vi "HFRR ADV v040.vi"() -> ()   [LabVIEW 2025] (continued)
        n290 = Format Into String(format string="%<%I:%M:%S:%p %d:%B:%Y>T", w374) -> (resulting string=→"Time Stamp":string)  [unwired: 2 in, 1 out]
        n291 = local read "Service Password enable"() -> (w366:bool)
        n292 = local read "FILE"() -> (w371:string)
        n293 = call <vilib>:"Trim Whitespace.vi"("string"=w371) -> ("trimmed string"=w370:string)  [unwired: 1 in]
        n294 = String Length(string=w370) -> (length=w369:i32)
        n295 = Greater?(x=w369, y=1) -> (0:w367:bool)
        n296 = case shown="False" w367 {
          tunnel: w366 -> [w395 _]
          frame False {
            n297 = case shown="False" w395 {
              frame True {
                w396 = "Test Start In Service Mode" ("Tip Strip")
                w397 = T19."Enabled" ("Disabled")
                n298 = property on="Auto Start Test" class="Bool (strict)"("DisabledEnum"=w397, "TipStrip"=w396) -> ()  [unwired: 2 in, 2 out]
                n299 = property on="RUN" class="Bool (strict)"("DisabledEnum"=w397, "TipStrip"=w396) -> ()  [unwired: 2 in, 2 out]
              }
              frame False {
                w398 = "Enter File Name to Start Test" ("Tip Strip")
                w399 = T19."Disabled and Grayed Out" ("Disabled")
                n300 = property on="Auto Start Test" class="Bool (strict)"("DisabledEnum"=w399, "TipStrip"=w398) -> ()  [unwired: 2 in, 2 out]
                n301 = property on="RUN" class="Bool (strict)"("DisabledEnum"=w399, "TipStrip"=w398) -> ()  [unwired: 2 in, 2 out]
              }
            }
          }
          frame True {
            w400 = "" ("Tip Strip")
            w401 = T19."Enabled" ("Disabled")
            n302 = property on="Auto Start Test" class="Bool (strict)"("DisabledEnum"=w401, "TipStrip"=w400) -> ()  [unwired: 2 in, 2 out]
            n303 = property on="RUN" class="Bool (strict)"("DisabledEnum"=w401, "TipStrip"=w400) -> ()  [unwired: 2 in, 2 out]
          }
        }
      }
      event "RUN": Value Change {
        n304 = event-data() -> ()  [unwired: 1 in, 6 out]
        n305 = local read "RUN"() -> (w403:bool)
        n306 = case shown="False" w403 {
          frame False {
            n307 = flat-sequence {
              frame #0 {
                n308 = local write "START TEMP"(FALSE ("START TEMP")) -> ()
              }
              frame #1 {
                n309 = Wait (ms)(milliseconds to wait=u32 1500) -> ()  [unwired: 1 out]
              }
              frame #2 {
                n310 = local write "Humidity 2"(TRUE ("Humidity")) -> ()
              }
              frame #3 {
                n311 = local write "Due Write"("VC;0") -> ()
              }
              frame #4 {
                n312 = Wait (ms)(milliseconds to wait=u32 1500) -> ()  [unwired: 1 out]
              }
              frame #5 {
                w413 = T19."Enabled" ("Disabled")
                (unwired) T26."Imaging" ("Main Dashboard Buttons")
                (unwired) T21."Adv Scar" ("Main Tab")
                w415 = "" ("FILE")
                n313 = local write "measured_stroke"(0.0 ("measured_stroke")) -> ()
                n314 = local write "Due Write"("VC;0") -> ()
                n315 = local write "FILE"(w415) -> ()
                n316 = local write "Batch Ref Num :"(w415) -> ()
                n317 = local write "Fuel Discription :"(w415) -> ()
                n318 = local write "Main Tab"(T2."Adv Scar" ("Main Tab")) -> ()
                n319 = local write "Remarks :"(w415) -> ()
                n320 = local write "Main Dashboard Buttons"(T1."Imaging" ("Main Dashboard Buttons")) -> ()
                n321 = local write "TEST FILE NAM,E SAVED"(FALSE ("TEST FILE NAM,E SAVED")) -> ()
                n322 = property on="Stroke ( mm )" class="WFChart (strict)"("History Data"=cluster{"y":dbl, dbl, "y":dbl}[] []) -> ()  [unwired: 2 in, 2 out]
                n323 = property on="Auto Start Test" class="Bool (strict)"("Visible"=TRUE) -> ()  [unwired: 2 in, 2 out]
                n324 = property on="FRICVALZ 2" class="Bool (strict)"("DisabledEnum"=w413) -> ()  [unwired: 2 in, 2 out]
                n325 = property on="FRICVALZ 4" class="Bool (strict)"("DisabledEnum"=w413) -> ()  [unwired: 2 in, 2 out]
                n326 = property on="FRICVALZ 3" class="Bool (strict)"("DisabledEnum"=w413) -> ()  [unwired: 2 in, 2 out]
              }
            }
          }
          frame True {
            n327 = stacked-sequence {
              frame #0 {
                n328 = local write "Due Write"("DAC;200") -> ()
              }
              frame #1 {
                n329 = Wait (ms)(milliseconds to wait=u32 1500) -> ()  [unwired: 1 out]
              }
              frame #2 {
                n330 = local write "Due Write"("DAC;200") -> ()
              }
              frame #3 {
                n331 = Wait (ms)(milliseconds to wait=u32 1500) -> ()  [unwired: 1 out]
              }
              frame #4 {
                n332 = local write "Due Write"("VC;1") -> ()
              }
              frame #5 {
                n333 = Wait (ms)(milliseconds to wait=u32 2000) -> ()  [unwired: 1 out]
              }
              frame #6 {
                n334 = local write "Due Write"("VC;1") -> ()
              }
              frame #7 {
                n335 = Wait (ms)(milliseconds to wait=u32 2000) -> ()  [unwired: 1 out]
              }
              frame #8 {
                w427 = T19."Disabled" ("Disabled")
                n336 = property on="Auto Start Test" class="Bool (strict)"("Visible"=FALSE) -> ()  [unwired: 2 in, 2 out]
                n337 = local write "START TEMP"(TRUE ("START TEMP")) -> ()
                n338 = property on="FRICVALZ 2" class="Bool (strict)"("DisabledEnum"=w427) -> ()  [unwired: 2 in, 2 out]
                n339 = property on="FRICVALZ 4" class="Bool (strict)"("DisabledEnum"=w427) -> ()  [unwired: 2 in, 2 out]
                n340 = property on="FRICVALZ 3" class="Bool (strict)"("DisabledEnum"=w427) -> ()  [unwired: 2 in, 2 out]
              }
            }
          }
        }
      }
      event "run test Calibration": Value Change {
        n341 = event-data() -> ()  [unwired: 1 in, 6 out]
        n342 = local read "run test Calibration"() -> (w429:bool)
        n343 = case shown="True" w429 {
          frame False {
            n344 = flat-sequence {
              frame #0 {
                n345 = local write "START TEMP"(FALSE ("START TEMP")) -> ()
              }
              frame #1 {
                n346 = Wait (ms)(milliseconds to wait=u32 1500) -> ()  [unwired: 1 out]
              }
              frame #2 {
              }
              frame #3 {
                n347 = local write "Due Write"("VC;0") -> ()
              }
              frame #4 {
                n348 = Wait (ms)(milliseconds to wait=u32 1500) -> ()  [unwired: 1 out]
              }
              frame #5 {
                n349 = local write "Due Write"("VC;0") -> ()
              }
            }
          }
          frame True {
            n350 = flat-sequence {
              frame #0 {
                n351 = local write "Due Write"("VC;1") -> ()
              }
              frame #1 {
                n352 = Wait (ms)(milliseconds to wait=u32 2000) -> ()  [unwired: 1 out]
              }
              frame #2 {
                n353 = local write "Due Write"("VC;1") -> ()
              }
              frame #3 {
                n354 = Wait (ms)(milliseconds to wait=u32 2000) -> ()  [unwired: 1 out]
              }
              frame #4 {
                n355 = local write "START TEMP"(TRUE ("START TEMP")) -> ()
              }
            }
          }
        }
      }
      event "Auto": Value Change {
        n356 = event-data() -> ()  [unwired: 1 in, 6 out]
        n357 = stacked-sequence {
          frame #0 {
            n358 = local write "FILE"("") -> ()
          }
          frame #1 {
            n359 = Get Date/Time In Seconds() -> (seconds since 1Jan1904=w445:timestamp)
            n360 = Format Into String(format string="%<%I_%M_%S_%p_%d_%B_%Y>T", w445) -> (resulting string=w444:string)  [unwired: 2 in, 1 out]
            n361 = local write "FILE"(w444) -> ()
          }
        }
        n362 = local read "Auto"() -> (w442:bool)
        n363 = Not(x=w442) -> (.not. x?=w441:bool)
        n364 = local write "Auto"(w441) -> ()
      }
      event "Auto Start Temp": Value Change {
        n365 = event-data() -> ()  [unwired: 1 in, 6 out]
        n366 = local read "Auto Start Test"() -> (w448:bool)
        n367 = case shown="False" w448 {
          frame False {
            n368 = stacked-sequence {
              frame #0 {
                n369 = local write "START TEMP"(FALSE ("START TEMP")) -> ()
              }
              frame #1 {
                n370 = Wait (ms)(milliseconds to wait=u32 2000) -> ()  [unwired: 1 out]
              }
              frame #2 {
                n371 = local write "Due Write"("VC;0") -> ()
              }
              frame #3 {
                n372 = Wait (ms)(milliseconds to wait=u32 2000) -> ()  [unwired: 1 out]
              }
              frame #4 {
                w459 = T19."Enabled" ("Disabled")
                (unwired) T26."Imaging" ("Main Dashboard Buttons")
                w460 = "" ("FILE")
                n373 = local write "Main Tab"(T2."Adv Scar" ("Main Tab")) -> ()
                n374 = local write "measured_stroke"(0.0 ("measured_stroke")) -> ()
                n375 = local write "Main Dashboard Buttons"(T1."Imaging" ("Main Dashboard Buttons")) -> ()
                n376 = property on="RUN" class="Bool (strict)"("Visible"=TRUE) -> ()  [unwired: 2 in, 2 out]
                n377 = local write "Due Write"("VC;0") -> ()
                n378 = local write "Humidity 2"(TRUE ("Humidity")) -> ()
                n379 = local write "TEST FILE NAM,E SAVED"(FALSE ("TEST FILE NAM,E SAVED")) -> ()
                n380 = local write "Fuel Discription :"(w460) -> ()
                n381 = local write "Batch Ref Num :"(w460) -> ()
                n382 = local write "Remarks :"(w460) -> ()
                n383 = local write "FILE"(w460) -> ()
                n384 = property on="FRICVALZ 2" class="Bool (strict)"("DisabledEnum"=w459) -> ()  [unwired: 2 in, 2 out]
                n385 = property on="FRICVALZ 4" class="Bool (strict)"("DisabledEnum"=w459) -> ()  [unwired: 2 in, 2 out]
                n386 = property on="FRICVALZ 3" class="Bool (strict)"("DisabledEnum"=w459) -> ()  [unwired: 2 in, 2 out]
              }
            }
          }
          frame True {
            n387 = stacked-sequence {
              frame #0 {
                n388 = local write "Due Write"("DAC;200") -> ()
              }
              frame #1 {
                n389 = Wait (ms)(milliseconds to wait=u32 1500) -> ()  [unwired: 1 out]
              }
              frame #2 {
                n390 = local write "Due Write"("DAC;200") -> ()
              }
              frame #3 {
                n391 = Wait (ms)(milliseconds to wait=u32 1000) -> ()  [unwired: 1 out]
              }
              frame #4 {
                n392 = local write "Due Write"("VC;1") -> ()
              }
              frame #5 {
                n393 = Wait (ms)(milliseconds to wait=u32 2000) -> ()  [unwired: 1 out]
              }
              frame #6 {
                n394 = local write "Due Write"("VC;1") -> ()
              }
              frame #7 {
                n395 = Wait (ms)(milliseconds to wait=u32 2000) -> ()  [unwired: 1 out]
              }
              frame #8 {
                w471 = T19."Disabled" ("Disabled")
                n396 = property on="RUN" class="Bool (strict)"("Visible"=FALSE) -> ()  [unwired: 2 in, 2 out]
                n397 = property on="FRICVALZ 2" class="Bool (strict)"("DisabledEnum"=w471) -> ()  [unwired: 2 in, 2 out]
                n398 = property on="FRICVALZ 4" class="Bool (strict)"("DisabledEnum"=w471) -> ()  [unwired: 2 in, 2 out]
                n399 = property on="FRICVALZ 3" class="Bool (strict)"("DisabledEnum"=w471) -> ()  [unwired: 2 in, 2 out]
                "START TEMP" <- TRUE
              }
            }
          }
        }
      }
      event "FILE", "USERNAME", "USER ID": Mouse Enter {
        n400 = event-data() -> ()  [unwired: 1 in, 4 out]
        n401 = dll-call lib="kernel32.dll" fn="Wow64DisableWow64FsRedirection"("OldValue"=0) -> (error out=w478:errorcluster, "OldValue"=w476:i32)  [unwired: 4 in, 1 out]
        n402 = call <vilib>:"System Exec.vi"("run minimized? (F)"=TRUE, "error in (no error)"=w478, "command line"="C:\\Program Files\\Common Files\\Microsoft Shared\\Ink\\TabTip.exe") -> ("error out"=w477:errorcluster)  [unwired: 5 in, 3 out]
        n403 = dll-call lib="kernel32.dll" fn="Wow64EnableWow64FsRedirection"(error in=w477, "OldValue"=w476) -> ()  [unwired: 4 in, 2 out]
      }
      event "EDIT": Value Change {
        n404 = event-data() -> ()  [unwired: 1 in, 6 out]
        n405 = local read "EDIT"() -> (w479:bool)
        n406 = case shown="False" w479 {
          frame False {
            n407 = control-ref of="This VI"() -> (w496:refnum<vi>)
            n408 = property class="VI"(reference=w496) -> (reference out=w487:refnum<vi>, error out=w491:errorcluster, "Panel"=w495:refnum<vi>)  [unwired: 1 in]
            n409 = property class="Pnl"(reference=w495, error in=w491) -> (reference out=w489:refnum<vi>, error out=w492:errorcluster, "Panes[]"=w494:refnum<vi>[])
            n410 = for {
              tunnel: w494 -> [w502] mode=indexing
              tunnel: T24."Always Off" ("Horizontal Scrollbar Visibility") -> [w501]
              tunnel: w492 -> [w498]
              tunnel: [w497] -> w490
              n411 = property class="Pane"(reference=w502, error in=w498, "HorizScrollbarVisibility"=w501) -> (reference out=w499:refnum<vi>, error out=w500:errorcluster)
              n412 = Close Reference(reference=w499, error in (no error)=w500) -> (error out=w497:errorcluster)
            }
            n413 = Close Reference(reference=w489, error in (no error)=w490) -> (error out=w488:errorcluster)
            n414 = Close Reference(reference=w487, error in (no error)=w488) -> (error out=w482:errorcluster)
            "error out 7" <- w482
            n415 = call <vilib>:"Clear Errors.vi"("error in (no error)"=w482) -> ("error out"=w481:errorcluster)  [unwired: 5 in, 1 out]
            n416 = local write "Service Password enable"(FALSE ("Service Password enable")) -> ()
            n417 = call <userlib>:"Fit VI window to Largest Dec.vi"("error in (no error)"=w481, "border spacing (2 px)"=1) -> ("error out"=w486:errorcluster, "dup VI Ref"=w484:refnum<vi>)  [unwired: 4 in]
            n418 = invoke on="Invoke Node" class="VI" method="FP.Run-Time Position.Maximized"(reference=w484, error in=w486) -> (error out=w485:errorcluster)  [unwired: 2 in, 3 out]
            n419 = call <vilib>:"Clear Errors.vi"("error in (no error)"=w485) -> ()  [unwired: 5 in, 2 out]
          }
          frame True {
          }
        }
      }
      event "Heater Button": Value Change {
        n420 = event-data() -> ()  [unwired: 1 in, 6 out]
        n421 = local read "Heater Button"() -> (w503:bool)
        n422 = case shown="True" w503 {
          frame True {
            n423 = stacked-sequence {
              frame #0 {
                n424 = Wait (ms)(milliseconds to wait=u32 1500) -> ()  [unwired: 1 out]
              }
              frame #1 {
                n425 = local read "Set Temp"() -> (w505:dbl)
                n426 = Number To Fractional String(number=w505, precision (6)=i16 2) -> (F-format string=w508:string)  [unwired: 2 in]
                n427 = Concatenate Strings("ST;" ("Command"), w508) -> (w507:string)
                n428 = local write "Due Write"(w507) -> ()
              }
              frame #2 {
                n429 = Wait (ms)(milliseconds to wait=u32 1500) -> ()  [unwired: 1 out]
              }
              frame #3 {
                n430 = local write "Due Write"("HE;1" ("Command")) -> ()
              }
              frame #4 {
                n431 = Wait (ms)(milliseconds to wait=u32 1500) -> ()  [unwired: 1 out]
              }
              frame #5 {
                n432 = stacked-sequence {
                  frame #0 {
                    n433 = Wait (ms)(milliseconds to wait=u32 1500) -> ()  [unwired: 1 out]
                  }
                  frame #1 {
                    n434 = local read "Set Temp"() -> (w514:dbl)
                    n435 = Number To Fractional String(number=w514, precision (6)=i16 2) -> (F-format string=w517:string)  [unwired: 2 in]
                    n436 = Concatenate Strings("ST;" ("Command"), w517) -> (w516:string)
                    n437 = local write "Due Write"(w516) -> ()
                  }
                  frame #2 {
                    n438 = Wait (ms)(milliseconds to wait=u32 1500) -> ()  [unwired: 1 out]
                  }
                  frame #3 {
                    n439 = local write "Due Write"("HE;1" ("Command")) -> ()
                  }
                  frame #4 {
                    n440 = Wait (ms)(milliseconds to wait=u32 1500) -> ()  [unwired: 1 out]
                  }
                }
              }
            }
          }
          frame False {
            n441 = stacked-sequence {
              frame #0 {
                n442 = Wait (ms)(milliseconds to wait=u32 1500) -> ()  [unwired: 1 out]
              }
              frame #1 {
                n443 = Concatenate Strings("ST;" ("Command"), "0" ("string")) -> (w524:string)
                n444 = local write "Due Write"(w524) -> ()
              }
              frame #2 {
                n445 = Wait (ms)(milliseconds to wait=u32 1500) -> ()  [unwired: 1 out]
              }
              frame #3 {
                n446 = local write "Due Write"("HE;0" ("Command")) -> ()
              }
              frame #4 {
                n447 = Wait (ms)(milliseconds to wait=u32 1500) -> ()  [unwired: 1 out]
              }
            }
          }
        }
      }
      event "Headen Service Button": Value Change {
        n448 = event-data() -> ()  [unwired: 1 in, 6 out]
        n449 = local read "Headen Service Button"() -> (w529:bool)
        n450 = case shown="True" w529 {
          frame False {
            n451 = property on="Password 3" class="Clust (strict)"("Visible"=FALSE) -> ()  [unwired: 2 in, 2 out]
            n452 = property on="Service Password Log" class="Str"("Visible"=FALSE) -> ()  [unwired: 2 in, 2 out]
          }
          frame True {
            n453 = property on="Password 3" class="Clust (strict)"("Visible"=TRUE) -> ()  [unwired: 2 in, 2 out]
            n454 = property on="Service Password Log" class="Str"("Visible"=TRUE) -> ()  [unwired: 2 in, 2 out]
          }
        }
      }
      event "Password 3.Service Password": Value Change {
        n455 = event-data() -> ()  [unwired: 1 in, 6 out]
        n456 = Unbundle By Name("Password 3") -> ("Service Password"=w536:string)
        n457 = call <vilib>:"Trim Whitespace.vi"("string"=w536) -> ("trimmed string"=w534:string)  [unwired: 1 in]
        n458 = Equal?(x=w534, y="Service@123") -> (x = y?=w535:bool)
        n459 = case shown="False" w535 {
          selector: w535 -> [w539 w541]
          frame False {
            n460 = local write "Service Password enable"(w539) -> ()
            n461 = property on="Service Password Log" class="Str"("Visible"=TRUE) -> ()  [unwired: 2 in, 2 out]
          }
          frame True {
            n462 = property on="Service Password Log" class="Str"("Visible"=FALSE) -> ()  [unwired: 2 in, 2 out]
            "Service Password enable" <- w541
          }
        }
      }
      event "Sign In": Value Change {
        w543 = FALSE ("Visible")
        n463 = event-data() -> ()  [unwired: 1 in, 6 out]
        n464 = property on="About" class="Clust (strict)"("Visible"=w543) -> ()  [unwired: 2 in, 2 out]
        n465 = property on="Password 3" class="Clust (strict)"("Visible"=w543) -> ()  [unwired: 2 in, 2 out]
        n466 = property on="Service Password Log" class="Str"("Visible"=FALSE) -> ()  [unwired: 2 in, 2 out]
      }
      event "Info": Value Change {
        n467 = event-data() -> ()  [unwired: 1 in, 6 out]
        n468 = local read "Info"() -> (w545:bool)
        n469 = case shown="False" w545 {
          frame False {
            n470 = property on="About" class="Clust (strict)"("Visible"=FALSE) -> ()  [unwired: 2 in, 2 out]
          }
          frame True {
            n471 = property on="About" class="Clust (strict)"("Visible"=TRUE) -> ()  [unwired: 2 in, 2 out]
          }
        }
      }
      event "Calibration": Value Change {
        n472 = event-data() -> ()  [unwired: 1 in, 6 out]
        n473 = local read "Calibration"() -> (w549:bool)
        n474 = case shown="False" w549 {
          frame False {
            n475 = property on="Calibration 2" class="TabCtl (strict)"("Visible"=FALSE) -> ()  [unwired: 2 in, 2 out]
            n476 = local write "Cal Password"("" ("Cal Password")) -> ()
          }
          frame True {
            n477 = property on="Calibration 2" class="TabCtl (strict)"("Visible"=TRUE) -> ()  [unwired: 2 in, 2 out]
            n478 = local write "Cal Password"("" ("Cal Password")) -> ()
          }
        }
        n479 = property on="Wrong Password" class="Str"("Visible"=FALSE) -> ()  [unwired: 2 in, 2 out]
      }
      event "Cal Password": Value Change {
        n480 = event-data() -> ()  [unwired: 1 in, 6 out]
        n481 = local read "Cal Password"() -> (w557:string)
        n482 = call <vilib>:"Trim Whitespace.vi"("string"=w557) -> ("trimmed string"=w556:string)  [unwired: 1 in]
        n483 = Equal?(x=w556, y="Cal@321") -> (x = y?=w554:bool)
        n484 = case shown="True" w554 {
          frame False {
            n485 = property on="Wrong Password" class="Str"("Visible"=TRUE) -> ()  [unwired: 2 in, 2 out]
          }
          frame True {
            n486 = property on="Wrong Password" class="Str"("Visible"=FALSE) -> ()  [unwired: 2 in, 2 out]
            n487 = local write "Main Tab"(T2."About" ("Main Tab")) -> ()
            n488 = local write "Cal Password"("" ("Cal Password")) -> ()
            n489 = local write "Main Dashboard Buttons"(T1."About" ("Main Dashboard Buttons")) -> ()
            n490 = property on="Calibration 2" class="TabCtl (strict)"("Visible"=FALSE) -> ()  [unwired: 2 in, 2 out]
            n491 = local write "Calibration"(FALSE ("Calibration")) -> ()
          }
        }
      }
      event "Calibration Selection": Value Change {
        n492 = event-data() -> ()  [unwired: 1 in, 6 out]
        n493 = local read "Calibration Selection"() -> (w566:T8)
        n494 = case shown="\"Stroke Calibration\"" w566 {
          tunnel: [T7."Stroke" ("Main Calibration Tab") T7."Friction" ("Main Calibration Tab") T7."Main" ("Main Calibration Tab") T7."Temperature" ("Main Calibration Tab")] -> w565
          frame "Stroke Calibration" {
          }
          frame "Friction Force Calibration" {
          }
          frame Default {
          }
          frame "Temperature Calibration" {
          }
        }
        n495 = local write "Main Calibration Tab"(w565) -> ()
      }
      event "Back Stroke": Value Change {
        n496 = event-data() -> ()  [unwired: 1 in, 6 out]
        n497 = local write "Main Stroke Tab"(T9."Step 1" ("Main Stroke Tab")) -> ()
        n498 = local write "Main Calibration Tab"(T7."Main" ("Main Calibration Tab")) -> ()
        n499 = local write "Back Stroke"(FALSE ("Back Stroke")) -> ()
        n500 = local write "Calibration Selection"(T8."Default" ("Calibration Selection")) -> ()
      }
      event "Step 2 Back": Value Change {
        n501 = event-data() -> ()  [unwired: 1 in, 6 out]
        n502 = local write "Main Stroke Tab"(T9."Step 1" ("Main Stroke Tab")) -> ()
        n503 = local write "Step 2 Back"(FALSE ("Back Stroke")) -> ()
        n504 = local write "Calibration Selection"(T8."Default" ("Calibration Selection")) -> ()
      }
      event "Step 3 Back": Value Change {
        n505 = event-data() -> ()  [unwired: 1 in, 6 out]
        n506 = local write "Main Stroke Tab"(T9."Step 2" ("Main Stroke Tab")) -> ()
        n507 = local write "Step 3 Back"(FALSE ("Back Stroke")) -> ()
        n508 = local write "Calibration Selection"(T8."Default" ("Calibration Selection")) -> ()
      }
      event "Step 4 Back": Value Change {
        n509 = event-data() -> ()  [unwired: 1 in, 6 out]
        n510 = local write "Main Stroke Tab"(T9."Step 3" ("Main Stroke Tab")) -> ()
        n511 = local write "Step 4 Back"(FALSE ("Back Stroke")) -> ()
        n512 = local write "Calibration Selection"(T8."Default" ("Calibration Selection")) -> ()
      }
      event "Step 5 Back": Value Change {
        n513 = event-data() -> ()  [unwired: 1 in, 6 out]
        n514 = local write "Main Stroke Tab"(T9."Step 4" ("Main Stroke Tab")) -> ()
        n515 = local write "Step 5 Back"(FALSE ("Back Stroke")) -> ()
        n516 = local write "Calibration Selection"(T8."Default" ("Calibration Selection")) -> ()
      }
      event "Step 6 Back": Value Change {
        n517 = event-data() -> ()  [unwired: 1 in, 6 out]
        n518 = local write "Main Stroke Tab"(T9."Step 5" ("Main Stroke Tab")) -> ()
        n519 = local write "Step 6 Back"(FALSE ("Back Stroke")) -> ()
        n520 = local write "Calibration Selection"(T8."Default" ("Calibration Selection")) -> ()
      }
      event "Back Stroke step 7": Value Change {
        n521 = event-data() -> ()  [unwired: 1 in, 6 out]
        n522 = local write "Main Stroke Tab"(T9."Step 5" ("Main Stroke Tab")) -> ()
        n523 = local write "Back Stroke step 7"(FALSE ("Back Stroke")) -> ()
        n524 = local write "Calibration Selection"(T8."Default" ("Calibration Selection")) -> ()
      }
      event "Back Stroke step 8": Value Change {
        n525 = event-data() -> ()  [unwired: 1 in, 6 out]
        n526 = local write "Main Stroke Tab"(T9."Step 7" ("Main Stroke Tab")) -> ()
        n527 = local write "Back Stroke step 8"(FALSE ("Back Stroke")) -> ()
        n528 = local write "Calibration Selection"(T8."Default" ("Calibration Selection")) -> ()
      }
      event "Back Stroke 8": Value Change {
        n529 = event-data() -> ()  [unwired: 1 in, 6 out]
        n530 = local write "MOVE CARRIAGE TO"(0.2 ("MOVE CARRIAGE TO")) -> ()
        n531 = local write "Main Stroke Tab"(T9."Step 1" ("Main Stroke Tab")) -> ()
        n532 = local write "Calibration Selection"(T8."Default" ("Calibration Selection")) -> ()
        n533 = local write "Back Stroke 8"(FALSE ("Back Stroke 8")) -> ()
      }
      event "Continue Stroke": Value Change {
        n534 = event-data() -> ()  [unwired: 1 in, 6 out]
        n535 = local write "Main Stroke Tab"(T9."Step 2" ("Main Stroke Tab")) -> ()
        n536 = local write "Continue Stroke"(FALSE ("Continue Stroke")) -> ()
      }
      event "Continue Stroke step 2": Value Change {
        n537 = event-data() -> ()  [unwired: 1 in, 6 out]
        n538 = local write "Main Stroke Tab"(T9."Step 3" ("Main Stroke Tab")) -> ()
        n539 = local write "Continue Stroke step 2"(FALSE ("Continue Stroke")) -> ()
      }
      event "Continue Stroke step 3": Value Change {
        n540 = event-data() -> ()  [unwired: 1 in, 6 out]
        n541 = local write "Main Stroke Tab"(T9."Step 4" ("Main Stroke Tab")) -> ()
        n542 = local write "Continue Stroke step 3"(FALSE ("Continue Stroke")) -> ()
      }
      event "Continue Stroke step 4": Value Change {
        n543 = event-data() -> ()  [unwired: 1 in, 6 out]
        n544 = local write "Main Stroke Tab"(T9."Step 5" ("Main Stroke Tab")) -> ()
        n545 = local write "Continue Stroke step 4"(FALSE ("Continue Stroke")) -> ()
      }
      event "Continue Stroke step 5": Value Change {
        n546 = event-data() -> ()  [unwired: 1 in, 6 out]
        n547 = local write "Main Stroke Tab"(T9."Step 7" ("Main Stroke Tab")) -> ()
        n548 = local write "Continue Stroke step 5"(FALSE ("Continue Stroke")) -> ()
      }
      event "Continue Stroke step 6": Value Change {
        n549 = event-data() -> ()  [unwired: 1 in, 6 out]
        n550 = local write "Main Stroke Tab"(T9."Step 7" ("Main Stroke Tab")) -> ()
        n551 = local write "Continue Stroke step 6"(FALSE ("Continue Stroke")) -> ()
      }
      event "Continue Stroke step 7": Value Change {
        w614 = FALSE ("0.2mm")
        n552 = event-data() -> ()  [unwired: 1 in, 6 out]
        n553 = local write "0.4 mm"(w614) -> ()
        n554 = local write "0.6 mm"(w614) -> ()
        n555 = local write "1.0 mm"(w614) -> ()
        n556 = local write "1.2 mm"(w614) -> ()
        n557 = local write "0.2 2"(w614) -> ()
        n558 = local write "0.4 2"(w614) -> ()
        n559 = local write "0.6 2"(w614) -> ()
        n560 = local write "0.8 2"(w614) -> ()
        n561 = local write "1.0 2"(w614) -> ()
        n562 = local write "1.2"(w614) -> ()
        n563 = local write "0.2mm"(w614) -> ()
        n564 = local write "0.8mm"(w614) -> ()
        n565 = local write "Main Stroke Tab"(T9."Step 8" ("Main Stroke Tab")) -> ()
        n566 = local write "Continue Stroke step 7"(FALSE ("Continue Stroke")) -> ()
        n567 = local write "Stroke Test Complete"(T10."Test Progress" ("Stroke Test Complete")) -> ()
        "Position Measurment Temp" <- 4.0 ("Position Measurment Temp")
        "Calibration Tare" <- TRUE ("Calibration Tare")
        "MOVE CARRIAGE TO" <- 1.0 ("MOVE CARRIAGE TO")
      }
      event "Continue Stroke step 8": Value Change {
        n568 = event-data() -> ()  [unwired: 1 in, 6 out]
        n569 = local read "LVDT STROKE  Calibration"() -> (w619:dbl)
        n570 = local read "Position Measurment Temp"() -> (w620:dbl)
        n571 = case shown="0, Default" w620 {
          selector: w620 -> [w625 w630 w635 w640 _ w648 w651 w652]
          tunnel: w619 -> [w621 w626 w631 w636 w642 w645 _ _]
          frame 0, Default {
            w623 = TRUE ("0.2mm")
            n572 = Increment(x=w625) -> (x+1=w624:i32)
            n573 = local write "Position Measurment Temp"(w624) -> ()
            n574 = local write "0.2mm"(w623) -> ()
            n575 = local write "0.2 2"(w623) -> ()
            n576 = local write "MOVE CARRIAGE TO"(1.0 ("MOVE CARRIAGE TO")) -> ()
            "Calibration 0.2" <- w621
          }
          frame 1 {
            w628 = TRUE ("0.4 mm")
            n577 = Increment(x=w630) -> (x+1=w629:i32)
            n578 = local write "Calibration 0.4"(w626) -> ()
            n579 = local write "Position Measurment Temp"(w629) -> ()
            n580 = local write "0.4 mm"(w628) -> ()
            n581 = local write "MOVE CARRIAGE TO"(0.6 ("MOVE CARRIAGE TO")) -> ()
            n582 = local write "0.4 2"(w628) -> ()
          }
          frame 2 {
            w633 = TRUE ("0.6 mm")
            n583 = Increment(x=w635) -> (x+1=w634:i32)
            n584 = local write "Calibration 0.6"(w631) -> ()
            n585 = local write "Position Measurment Temp"(w634) -> ()
            n586 = local write "0.6 2"(w633) -> ()
            n587 = local write "0.6 mm"(w633) -> ()
            n588 = local write "MOVE CARRIAGE TO"(0.8 ("MOVE CARRIAGE TO")) -> ()
          }
          frame 3 {
            w637 = TRUE ("0.6 mm")
            n589 = Increment(x=w640) -> (x+1=w639:i32)
            n590 = local write "Position Measurment Temp"(w639) -> ()
            n591 = local write "MOVE CARRIAGE TO"(1.0 ("MOVE CARRIAGE TO")) -> ()
            n592 = local write "0.8mm"(w637) -> ()
            n593 = local write "0.8 2"(w637) -> ()
            "Calibration 0.8" <- w636
          }
          frame 4 {
            w643 = TRUE ("0.6 mm")
            n594 = local write "Position Measurment Temp"(6.0 ("Position Measurment Temp")) -> ()
            n595 = local write "MOVE CARRIAGE TO"(1.0 ("MOVE CARRIAGE TO")) -> ()
            n596 = local write "1.0 mm"(w643) -> ()
            n597 = local write "1.0 2"(w643) -> ()
            "Calibration 1.0" <- w642
          }
          frame 5 {
            w646 = TRUE ("0.6 mm")
            n598 = Increment(x=w648) -> (x+1=w647:i32)
            n599 = local write "Position Measurment Temp"(w647) -> ()
            n600 = local write "1.2 mm"(w646) -> ()
            n601 = local write "1.2"(w646) -> ()
            "Calibration 1.2" <- w645
          }
          frame 6 {
            n602 = Increment(x=w651) -> (x+1=w650:i32)
            n603 = local write "Position Measurment Temp"(w650) -> ()
            n604 = local write "Stroke Test Complete"(T10."Stroke Points Completed" ("Stroke Test Complete")) -> ()
          }
          frame 7 {
            n605 = stacked-sequence {
              tunnel: w652 -> [w653 _ _]
              frame #0 {
                n606 = Increment(x=w653) -> (x+1=w654:i32)
                n607 = local write "Main Stroke Tab"(T9."Step 9" ("Main Stroke Tab")) -> ()
                n608 = local write "Position Measurment Temp"(w654) -> ()
                n609 = Insert Into Array(array=dbl[] [], new element #1=0.2 ("new element/subarray"), new element #2=0.4 ("new element/subarray"), new element #3=0.6 ("new element/subarray"), new element #4=0.8 ("new element/subarray"), new element #5=1.0 ("new element/subarray"), new element #6=1.2 ("new element/subarray")) -> (→"1D stroke":dbl[])  [unwired: 1 in]
                n610 = local read "Calibration 0.2"() -> (w661:dbl)
                n611 = local read "Calibration 0.4"() -> (w660:dbl)
                n612 = local read "Calibration 0.6"() -> (w659:dbl)
                n613 = local read "Calibration 0.8"() -> (w658:dbl)
                n614 = local read "Calibration 1.0"() -> (w657:dbl)
                n615 = local read "Calibration 1.2"() -> (w656:dbl)
                n616 = Insert Into Array(array=dbl[] [], new element #1=w661, new element #2=w660, new element #3=w659, new element #4=w658, new element #5=w657, new element #6=w656) -> (→"Calibrated Voltage Value":dbl[])  [unwired: 1 in]
              }
              frame #1 {
                n617 = local read "calibration values"() -> (w684:dbl[])
                n618 = local read "Calibrated Voltage Value"() -> (w686:dbl[])
                n619 = Index Array(array=w684, index #1=1 ("index"), index #2=3 ("index"), index #3=5 ("index"), index #4=7 ("index"), index #5=9 ("index"), index #6=11 ("index")) -> (element #1=w677:dbl, element #2=w676:dbl, element #3=w675:dbl, element #4=w674:dbl, element #5=w673:dbl, element #6=w672:dbl)
                n620 = local read "1D stroke"() -> (w687:dbl[])
                n621 = for {
                  tunnel: [w696] -> w685 mode=indexing
                  tunnel: w687 -> [w695] mode=indexing
                  tunnel: w686 -> [w694] mode=indexing
                  tunnel: w677 -> [w693]
                  tunnel: w676 -> [w692]
                  tunnel: w675 -> [w691]
                  tunnel: w674 -> [w690]
                  tunnel: w673 -> [w689]
                  tunnel: w672 -> [w688]
                  n622 = formula code="if (stroke == 0.2)\n{\n    if ((voltage >= REF_02 - 0.2) && (voltage <= REF_02 + 0.2))\n        status = 1;\n    else\n        status = 0;\n}\nelse if (stroke == 0.4)\n{\n    if ((voltage >= REF_04 - 0.2) && (voltage <= REF_04 + 0.2))\n        status = 1;\n    else\n        status = 0;\n}\nelse if (stroke == 0.6)\n{\n    if ((voltage >= REF_06 - 0.2) && (voltage <= REF_06 + 0.2))\n        status = 1;\n    else\n        status = 0;\n}\nelse if (stroke == 0.8)\n{\n    if ((voltage >= REF_08 - 0.2) && (voltage <= REF_08 + 0.2))\n        status = 1;\n    else\n        status = 0;\n}\nelse if (stroke == 1.0)\n{\n    if ((voltage >= REF_10 - 0.4) && (voltage <= REF_10 + 0.4))\n        status = 1;\n    else\n        status = 0;\n}\nelse if (stroke == 1.2)\n{\n    if ((voltage >= REF_12 - 0.2) && (voltage <= REF_12 + 0.2))\n        status = 1;\n    else\n        status = 0;\n}\nelse\n{\n    status = 0;\n}"("stroke"=w695, "voltage"=w694, "REF_02"=w693, "REF_04"=w692, "REF_06"=w691, "REF_08"=w690, "REF_10"=w689, "REF_12"=w688) -> ("status"=w696:dbl)
                }
                "Status" <- w685
              }
              frame #2 {
                w703 = 1.0
                n623 = local read "Status"() -> (w710:dbl[])
                n624 = Index Array(array=w710) -> (element #1=w709:dbl, element #2=w708:dbl, element #3=w707:dbl, element #4=w706:dbl, element #5=w705:dbl, element #6=w704:dbl)  [unwired: 6 in]
                n625 = Equal?(x=w708, y=w703) -> (x = y?=w701:bool)
                n626 = Equal?(x=w707, y=w703) -> (x = y?=w700:bool)
                n627 = Equal?(x=w706, y=w703) -> (x = y?=w699:bool)
                n628 = Equal?(x=w705, y=w703) -> (x = y?=w698:bool)
                n629 = Equal?(x=w704, y=w703) -> (x = y?=w697:bool)
                n630 = Equal?(x=w709, y=w703) -> (x = y?=w702:bool)
                n631 = case shown="True" w702 {
                  selector: w702 -> [w721 w722]
                  frame True {
                    n632 = local write "Point 1 - 0.2 mm"(w721) -> ()
                    n633 = property on="Point 1 - 0.2 mm" class="Bool"("Caption.Visible"=w721) -> ()  [unwired: 2 in, 2 out]
                  }
                  frame False {
                    n634 = local write "Point 1 - 0.2 mm"(w722) -> ()
                    n635 = property on="Point 1 - 0.2 mm" class="Bool"("Caption.Visible"=w722) -> ()  [unwired: 2 in, 2 out]
                  }
                }
                n636 = case shown="True" w701 {
                  selector: w701 -> [w719 w720]
                  frame True {
                    n637 = local write "Point 2 - 0.4 mm"(w719) -> ()
                    n638 = property on="Point 2 - 0.4 mm" class="Bool"("Caption.Visible"=w719) -> ()  [unwired: 2 in, 2 out]
                  }
                  frame False {
                    n639 = local write "Point 2 - 0.4 mm"(w720) -> ()
                    n640 = property on="Point 2 - 0.4 mm" class="Bool"("Caption.Visible"=w720) -> ()  [unwired: 2 in, 2 out]
                  }
                }
                n641 = case shown="True" w698 {
                  selector: w698 -> [w713 w714]
                  frame True {
                    n642 = local write "Point 5 - 1.0 mm"(w713) -> ()
                    n643 = property on="Point 5 - 1.0 mm" class="Bool"("Caption.Visible"=w713) -> ()  [unwired: 2 in, 2 out]
                  }
                  frame False {
                    n644 = local write "Point 5 - 1.0 mm"(w714) -> ()
                    n645 = property on="Point 5 - 1.0 mm" class="Bool"("Caption.Visible"=w714) -> ()  [unwired: 2 in, 2 out]
                  }
                }
                n646 = case shown="True" w700 {
                  selector: w700 -> [w717 w718]
                  frame True {
                    n647 = local write "Point 3 - 0.6 mm"(w717) -> ()
                    n648 = property on="Point 3 - 0.6 mm" class="Bool"("Caption.Visible"=w717) -> ()  [unwired: 2 in, 2 out]
                  }
                  frame False {
                    n649 = local write "Point 3 - 0.6 mm"(w718) -> ()
                    n650 = property on="Point 3 - 0.6 mm" class="Bool"("Caption.Visible"=w718) -> ()  [unwired: 2 in, 2 out]
                  }
                }
                n651 = case shown="True" w699 {
                  selector: w699 -> [w715 w716]
                  frame True {
                    n652 = local write "Point 4 - 0.8 mm"(w715) -> ()
                    n653 = property on="Point 4 - 0.8 mm" class="Bool"("Caption.Visible"=w715) -> ()  [unwired: 2 in, 2 out]
                  }
                  frame False {
                    n654 = local write "Point 4 - 0.8 mm"(w716) -> ()
                    n655 = property on="Point 4 - 0.8 mm" class="Bool"("Caption.Visible"=w716) -> ()  [unwired: 2 in, 2 out]
                  }
                }
                n656 = case shown="True" w697 {
                  selector: w697 -> [w711 w712]
                  frame True {
                    n657 = local write "Point 6 - 1.2 mm"(w711) -> ()
                    n658 = property on="Point 6 - 1.2 mm" class="Bool"("Caption.Visible"=w711) -> ()  [unwired: 2 in, 2 out]
                  }
                  frame False {
                    n659 = local write "Point 6 - 1.2 mm"(w712) -> ()
                    n660 = property on="Point 6 - 1.2 mm" class="Bool"("Caption.Visible"=w712) -> ()  [unwired: 2 in, 2 out]
                  }
                }
              }
            }
          }
        }
      }
      event "TEMPERATURE STEP Back 1", "TEMPERATURE STEP Back air Temp": Value Change {
        n661 = event-data() -> ()  [unwired: 1 in, 6 out]
        n662 = stacked-sequence {
          frame #0 {
            n663 = local write "Main Calibration Tab"(T7."Main" ("Main Calibration Tab")) -> ()
            n664 = local write "Temperature Selection"(T13."Default" ("Temperature Selection")) -> ()
          }
          frame #1 {
            n665 = Wait (ms)(milliseconds to wait=u32 1000) -> ()  [unwired: 1 out]
            n666 = local write "Calibration Selection"(T8."Default" ("Calibration Selection")) -> ()
          }
          frame #2 {
            n667 = local write "Due Write"("CAL;END" ("Command")) -> ()
          }
          frame #3 {
            n668 = Wait (ms)(milliseconds to wait=u32 2000) -> ()  [unwired: 1 out]
          }
          frame #4 {
            n669 = local write "Due Write"("CAL;END" ("Command")) -> ()
          }
        }
      }
      event "Temperature Continue Step 1": Value Change {
        n670 = event-data() -> ()  [unwired: 1 in, 6 out]
        n671 = stacked-sequence {
          frame #0 {
            n672 = Wait (ms)(milliseconds to wait=u32 1500) -> ()  [unwired: 1 out]
          }
          frame #1 {
            n673 = local write "Due Write"("CAL;START" ("Command")) -> ()
          }
          frame #2 {
            n674 = Wait (ms)(milliseconds to wait=u32 1500) -> ()  [unwired: 1 out]
          }
          frame #3 {
            n675 = local write "Due Write"("CAL;START" ("Command")) -> ()
          }
          frame #4 {
            n676 = Wait (ms)(milliseconds to wait=u32 2000) -> ()  [unwired: 1 out]
          }
          frame #5 {
          }
          frame #6 {
            n677 = Wait (ms)(milliseconds to wait=u32 2000) -> ()  [unwired: 1 out]
          }
          frame #7 {
            # "CAL;A1;<true_T>"
            n678 = local write "Due Write"("CAL;A1;0" ("Command")) -> ()
          }
          frame #8 {
            n679 = local write "Tab Control 4"(T12."Step 2" ("Tab Control 4")) -> ()
          }
        }
      }
      event "Temperature Continue Step air Step 1": Value Change {
        n680 = event-data() -> ()  [unwired: 1 in, 6 out]
        n681 = stacked-sequence {
          frame #0 {
            n682 = Wait (ms)(milliseconds to wait=u32 1500) -> ()  [unwired: 1 out]
          }
          frame #1 {
            n683 = local write "Due Write"("CAL;START" ("Command")) -> ()
          }
          frame #2 {
            n684 = Wait (ms)(milliseconds to wait=u32 1500) -> ()  [unwired: 1 out]
          }
          frame #3 {
            n685 = local write "Due Write"("CAL;START" ("Command")) -> ()
          }
          frame #4 {
            n686 = Wait (ms)(milliseconds to wait=u32 2000) -> ()  [unwired: 1 out]
          }
          frame #5 {
          }
          frame #6 {
            n687 = Wait (ms)(milliseconds to wait=u32 2000) -> ()  [unwired: 1 out]
          }
          frame #7 {
            # "CAL;A1;<true_T>"
            n688 = local write "Due Write"("CAL;A1;0" ("Command")) -> ()
          }
          frame #8 {
            n689 = local write "Tab Control 4"(T12."Air Step 2" ("Tab Control 4")) -> ()
          }
        }
      }
      event "Temperature Selection": Value Change {
        n690 = event-data() -> ()  [unwired: 1 in, 6 out]
        n691 = local read "Temperature Selection"() -> (w746:T13)
        n692 = case shown="\"Sample Temperature\"" w746 {
          frame "Air Temperature" {
            n693 = local write "Tab Control 4"(T12."Air Step 1" ("Tab Control 4")) -> ()
          }
          frame "Sample Temperature" {
            n694 = local write "Tab Control 4"(T12."Step 1" ("Tab Control 4")) -> ()
          }
          frame "Default", Default {
          }
        }
      }
      event "Temperature Continue Step 2": Value Change {
        n695 = event-data() -> ()  [unwired: 1 in, 6 out]
        n696 = stacked-sequence {
          frame #0 {
            n697 = stacked-sequence {
              frame #0 {
                n698 = Wait (ms)(milliseconds to wait=u32 1500) -> ()  [unwired: 1 out]
              }
              frame #1 {
                # "CAL;A1;<true_T>"
                n699 = local read "Sensor value"() -> (→"Sample 0deg temp":dbl)
                n700 = local write "Due Write"("CAL;A1;0" ("Command")) -> ()
              }
              frame #2 {
                n701 = Wait (ms)(milliseconds to wait=u32 1500) -> ()  [unwired: 1 out]
              }
              frame #3 {
                # "CAL;A1;<true_T>"
                n702 = local write "Due Write"("CAL;A1;0" ("Command")) -> ()
              }
              frame #4 {
              }
            }
          }
          frame #1 {
            n703 = local write "Tab Control 4"(T12."Step 3" ("Tab Control 4")) -> ()
          }
        }
      }
      event "Temperature Continue Air Step 2": Value Change {
        n704 = event-data() -> ()  [unwired: 1 in, 6 out]
        n705 = stacked-sequence {
          frame #0 {
            n706 = stacked-sequence {
              frame #0 {
                n707 = Wait (ms)(milliseconds to wait=u32 1000) -> ()  [unwired: 1 out]
              }
              frame #1 {
                # "CAL;A1;<true_T>"
                n708 = local write "Due Write"("CAL;A1;0" ("Command")) -> ()
              }
              frame #2 {
                n709 = Wait (ms)(milliseconds to wait=u32 1000) -> ()  [unwired: 1 out]
              }
              frame #3 {
                # "CAL;A1;<true_T>"
                n710 = local write "Due Write"("CAL;A1;0" ("Command")) -> ()
              }
              frame #4 {
                n711 = local read "Sensor value"() -> (→"Air 0deg temp":dbl)
              }
            }
          }
          frame #1 {
            n712 = local write "Tab Control 4"(T12."Air Step 3" ("Tab Control 4")) -> ()
          }
        }
      }
      event "Temperature Continue Step 3": Value Change {
        n713 = event-data() -> ()  [unwired: 1 in, 6 out]
        n714 = stacked-sequence {
          frame #0 {
            n715 = stacked-sequence {
              frame #0 {
                n716 = Wait (ms)(milliseconds to wait=u32 1500) -> ()  [unwired: 1 out]
              }
              frame #1 {
              }
              frame #2 {
              }
              frame #3 {
                # "CAL;A1;<true_T>"
                n717 = local write "Due Write"("CAL;A1;60" ("Command")) -> ()
              }
              frame #4 {
                n718 = Wait (ms)(milliseconds to wait=u32 1000) -> ()  [unwired: 1 out]
              }
              frame #5 {
                # "CAL;A1;<true_T>"
                n719 = local read "Sensor value"() -> (→"Sample 60deg temp":dbl)
                n720 = local write "Due Write"("CAL;A1;60" ("Command")) -> ()
              }
            }
          }
          frame #1 {
            n721 = local read "Sample 0deg temp"() -> (w775:dbl)
            n722 = local read "Sample 60deg temp"() -> (w774:dbl)
            n723 = Add(x=w774, y="Temperature diff") -> (x+y=w772:dbl)
            n724 = Subtract(x=w774, y="Temperature diff") -> (x-y=w771:dbl)
            n725 = Add(x=w775, y="Temperature diff") -> (x+y=w770:dbl)
            n726 = Subtract(x=w775, y="Temperature diff") -> (x-y=w769:dbl)
            n727 = In Range and Coerce(upper limit=w772, x=w774, lower limit=w771) -> (In Range?=w768:bool)  [unwired: 1 out]
            n728 = In Range and Coerce(upper limit=w770, x=w775, lower limit=w769) -> (In Range?=w767:bool)  [unwired: 1 out]
            n729 = And(x=w768, y=w767) -> (x .and. y?=w766:bool)
            n730 = case shown="True" w766 {
              frame False {
                n731 = property on="Accept & Save sample Temperature step 4" class="Bool (strict)"("DisabledEnum"=T19."Disabled" ("Disabled")) -> ()  [unwired: 2 in, 2 out]
                n732 = local write "Sample Temperature Calibration  2"(enum32{"True", "Fail"}."Fail" ("Sample Temperature Calibration  2")) -> ()
              }
              frame True {
                n733 = property on="Accept & Save sample Temperature step 4" class="Bool (strict)"("DisabledEnum"=T19."Enabled" ("Disabled")) -> ()  [unwired: 2 in, 2 out]
                n734 = local write "Sample Temperature Calibration  2"(enum32{"True", "Fail"}."True" ("Sample Temperature Calibration  2")) -> ()
              }
            }
          }
          frame #2 {
          }
          frame #3 {
          }
          frame #4 {
          }
          frame #5 {
          }
          frame #6 {
            # "CAL;END"
          }
          frame #7 {
          }
          frame #8 {
            # "CAL;END"
          }
          frame #9 {
            n735 = local write "Tab Control 4"(T12."Step 4" ("Tab Control 4")) -> ()
          }
        }
      }
      event "Accept & Save sample Temperature step 4": Value Change {
        n736 = event-data() -> ()  [unwired: 1 in, 6 out]
        n737 = stacked-sequence {
          frame #0 {
            n738 = local write "Due Write"("CAL;SAVE" ("Command")) -> ()
          }
          frame #1 {
            n739 = Wait (ms)(milliseconds to wait=u32 1000) -> ()  [unwired: 1 out]
          }
          frame #2 {
            n740 = local write "Due Write"("CAL;SAVE" ("Command")) -> ()
          }
          frame #3 {
            n741 = Wait (ms)(milliseconds to wait=u32 1000) -> ()  [unwired: 1 out]
          }
          frame #4 {
            n742 = local write "Due Write"("CAL;END" ("Command")) -> ()
          }
          frame #5 {
            n743 = Wait (ms)(milliseconds to wait=u32 1000) -> ()  [unwired: 1 out]
          }
          frame #6 {
            n744 = local write "Due Write"("CAL;END" ("Command")) -> ()
            n745 = local write "Temperature Selection"(T13."Default" ("Temperature Selection")) -> ()
            n746 = local write "Calibration Selection"(T8."Default" ("Calibration Selection")) -> ()
            n747 = local write "Tab Control 4"(T12."Main" ("Tab Control 4")) -> ()
            n748 = local write "Main Calibration Tab"(T7."Temperature" ("Main Calibration Tab")) -> ()
          }
        }
      }
      event "Accept & Save Air Temperature step 4": Value Change {
        n749 = event-data() -> ()  [unwired: 1 in, 6 out]
        n750 = stacked-sequence {
          frame #0 {
            n751 = local write "Due Write"("CAL;SAVE" ("Command")) -> ()
          }
          frame #1 {
            n752 = Wait (ms)(milliseconds to wait=u32 1000) -> ()  [unwired: 1 out]
          }
          frame #2 {
            n753 = local write "Due Write"("CAL;SAVE" ("Command")) -> ()
          }
          frame #3 {
            n754 = Wait (ms)(milliseconds to wait=u32 1000) -> ()  [unwired: 1 out]
          }
          frame #4 {
            n755 = local write "Due Write"("CAL;END" ("Command")) -> ()
          }
          frame #5 {
            n756 = Wait (ms)(milliseconds to wait=u32 1000) -> ()  [unwired: 1 out]
          }
          frame #6 {
            n757 = local write "Due Write"("CAL;END" ("Command")) -> ()
            n758 = local write "Tab Control 4"(T12."Main" ("Tab Control 4")) -> ()
            n759 = local write "Main Calibration Tab"(T7."Temperature" ("Main Calibration Tab")) -> ()
            n760 = local write "Temperature Selection"(T13."Default" ("Temperature Selection")) -> ()
            n761 = local write "Calibration Selection"(T8."Default" ("Calibration Selection")) -> ()
          }
        }
      }
      event "Temperature Continue Step 6": Value Change {
        n762 = event-data() -> ()  [unwired: 1 in, 6 out]
        n763 = stacked-sequence {
          frame #0 {
            n764 = stacked-sequence {
              frame #0 {
                n765 = Wait (ms)(milliseconds to wait=u32 1000) -> ()  [unwired: 1 out]
              }
              frame #1 {
              }
              frame #2 {
              }
              frame #3 {
                # "CAL;A1;<true_T>"
                n766 = local write "Due Write"("CAL;A1;60" ("Command")) -> ()
              }
              frame #4 {
                n767 = Wait (ms)(milliseconds to wait=u32 1000) -> ()  [unwired: 1 out]
              }
              frame #5 {
                # "CAL;A1;<true_T>"
                n768 = local write "Due Write"("CAL;A1;60" ("Command")) -> ()
              }
            }
          }
          frame #1 {
            n769 = local read "Sensor value"() -> (→"Air 60deg temp":dbl)
          }
          frame #2 {
          }
          frame #3 {
          }
          frame #4 {
          }
          frame #5 {
          }
          frame #6 {
            # "CAL;END"
          }
          frame #7 {
            n770 = local read "Temperature diff"() -> (w810:dbl)
            n771 = local read "Air 60deg temp"() -> (w809:dbl)
            n772 = local read "Air 0deg temp"() -> (w808:dbl)
            n773 = Add(x=w809, y=w810) -> (x+y=w817:dbl)
            n774 = Subtract(x=w809, y=w810) -> (x-y=w816:dbl)
            n775 = Add(x=w808, y=w810) -> (x+y=w815:dbl)
            n776 = Subtract(x=w808, y=w810) -> (x-y=w814:dbl)
            n777 = In Range and Coerce(upper limit=w817, x=w809, lower limit=w816) -> (In Range?=w813:bool)  [unwired: 1 out]
            n778 = In Range and Coerce(upper limit=w815, x=w808, lower limit=w814) -> (In Range?=w812:bool)  [unwired: 1 out]
            n779 = And(x=w813, y=w812) -> (x .and. y?=w811:bool)
            n780 = case shown="True" w811 {
              frame False {
                n781 = property on="Accept & Save Air Temperature step 4" class="Bool (strict)"("DisabledEnum"=T19."Disabled" ("Disabled")) -> ()  [unwired: 2 in, 2 out]
                n782 = local write "Sample Temperature Calibration"(enum32{"True", "Fail"}."Fail" ("Sample Temperature Calibration  2")) -> ()
              }
              frame True {
                n783 = local write "Sample Temperature Calibration"(enum32{"True", "Fail"}."True" ("Sample Temperature Calibration  2")) -> ()
                n784 = property on="Accept & Save Air Temperature step 4" class="Bool (strict)"("DisabledEnum"=T19."Enabled" ("Disabled")) -> ()  [unwired: 2 in, 2 out]
              }
            }
          }
          frame #8 {
            # "CAL;END"
          }
          frame #9 {
            n785 = local write "Tab Control 4"(T12."Air Step 4" ("Tab Control 4")) -> ()
          }
        }
      }
      event "Back Stroke step main temperature": Value Change {
        n786 = event-data() -> ()  [unwired: 1 in, 6 out]
        n787 = stacked-sequence {
          frame #0 {
            n788 = Wait (ms)(milliseconds to wait=u32 1000) -> ()  [unwired: 1 out]
          }
          frame #1 {
            # "CAL;END"
            n789 = local write "Due Write"("CAL;END" ("Command")) -> ()
          }
          frame #2 {
            n790 = Wait (ms)(milliseconds to wait=u32 1000) -> ()  [unwired: 1 out]
          }
          frame #3 {
            # "CAL;END"
            n791 = local write "Due Write"("CAL;END" ("Command")) -> ()
          }
          frame #4 {
            n792 = local write "Temperature Selection"(T13."Default" ("Temperature Selection")) -> ()
            n793 = local write "Calibration Selection"(T8."Default" ("Calibration Selection")) -> ()
            n794 = local write "Main Calibration Tab"(T7."Main" ("Main Calibration Tab")) -> ()
            n795 = local write "Tab Control 4"(T12."Main" ("Tab Control 4")) -> ()
          }
        }
      }
      event "TEMPERATURE STEP  Back 4", "TEMPERATURE STEP 1 Back 3", "TEMPERATURE STEP  Back 3", "TEMPERATURE STEP 1 Back 2", "Back Air TEMPERATURE Step 4", "Back SAMPLE TEMPERATURE Step 4": Value Change {
        # "Back Stroke step main temperature"
        n796 = event-data() -> ()  [unwired: 1 in, 6 out]
        n797 = stacked-sequence {
          frame #0 {
            n798 = Wait (ms)(milliseconds to wait=u32 1000) -> ()  [unwired: 1 out]
          }
          frame #1 {
            # "CAL;END"
            n799 = local write "Due Write"("CAL;END" ("Command")) -> ()
          }
          frame #2 {
            n800 = Wait (ms)(milliseconds to wait=u32 1000) -> ()  [unwired: 1 out]
          }
          frame #3 {
            # "CAL;END"
            n801 = local write "Due Write"("CAL;END" ("Command")) -> ()
          }
          frame #4 {
            # "TEMPERATURE STEP  Back 4"
            n802 = local write "Main Calibration Tab"(T7."Temperature" ("Main Calibration Tab")) -> ()
            n803 = local write "Temperature Selection"(T13."Default" ("Temperature Selection")) -> ()
            n804 = local write "Tab Control 4"(T12."Main" ("Tab Control 4")) -> ()
            n805 = local write "Calibration Selection"(T8."Default" ("Calibration Selection")) -> ()